vi "UHR-Fleezers Control (host) - 12.3.vi"() -> ()   [LabVIEW 2012] (continued)
                      n1986 = Square(x=w2941) -> (x^2=w2939:dbl)
                      n1987 = Square(x=w2940) -> (x^2=w2938:dbl)
                      n1988 = Add(x=w2939, y=w2938) -> (x+y=w2937:dbl)
                      n1989 = Square Root(x=w2937) -> (sqrt(x)=w2933:dbl)
                      n1990 = In Range and Coerce(upper limit="Limit Max (MHz)", x=w2933, lower limit="Limit Min (MHz)") -> (In Range?=w2926:bool)  [unwired: 1 out]
                      n1991 = Not(x="Limits Enable") -> (.not. x?=w2925:bool)
                      n1992 = Or(x=w2926, y=w2925) -> (x .or. y?=w2927:bool)
                      n1993 = case shown="True" w2927 {
                        tunnel: w2934 -> [_ w2967]
                        tunnel: w2933 -> [_ w2958]
                        tunnel: w2923 -> [_ w2965]
                        tunnel: w2932 -> [_ w2964]
                        tunnel: w2921 -> [_ w2963]
                        tunnel: w2931 -> [_ w2962]
                        tunnel: w2916 -> [_ w2960]
                        tunnel: w2915 -> [_ w2959]
                        frame False {
                        }
                        frame True {
                          n1994 = local read "BD 1 Frequency 3 (MHz)"() -> (w2966:dbl)
                          n1995 = local read "BD 2 Frequency 3 (MHz)"() -> (w2961:dbl)
                          n1996 = local write "Trap Delta (MHz)"(w2958) -> ()
                          n1997 = call "set RF board frequency - interlace.vi"("Board 2 Frequency Limits"=w2959, "Board 1 Frequency Limits"=w2960, "FPGA VI Reference In"=w2967, "Board 2 Frequency 3 (MHz)"=w2961, "Board 1 Frequency 3 (MHz)"=w2966, "Board 2 Frequency 2 (MHz)"=w2962, "Board 2 Frequency 1 (MHz)"=w2963, "Board 1 Frequency 2 (MHz)"=w2964, "Board 1 Frequency 1  (MHz)"=w2965) -> ()  [unwired: 1 in, 2 out]
                          n1998 = local write "BD 2 Frequency 1 (MHz)"(w2963) -> ()
                          n1999 = local write "BD 1 Frequency 1 (MHz)"(w2965) -> ()
                        }
                      }
                    }
                    frame True {
                    }
                  }
                }
                event Mouse Up {
                  n2000 = event-data() -> ("Button"=w2968:u16)  [unwired: 8 out]
                  n2001 = case shown="3" w2968 {
                    tunnel: [FALSE TRUE] -> w2969
                    frame 0, Default {
                    }
                    frame 3 {
                      n2002 = local read "Trap Delta (MHz)"() -> (w2971:dbl)
                      n2003 = property on="Initial delta (MHz)" class="DigNum (strict)"("Val(Sgnl)"=w2971) -> ()  [unwired: 2 in, 2 out]
                      n2004 = local write "Manipulating Trap"(FALSE ("Manipulating Trap")) -> ()
                    }
                  }
                }
              }
            }
          }
        }
      }
      event Mouse Move {
        n2005 = event-data() -> ()  [unwired: 6 out]
      }
    }
    n2006 = local read "Stop All"() -> (w2787:bool)
    n2007 = node-c288() -> ()  [unwired: 2 out]
  }
  n2008 = timed-loop "Main data acquisition loop (get data, process data for display, and save data to disk)" {
    tunnel: w7 -> [w3283]
    tunnel: w83 -> [w3282]
    tunnel: [w3312] -> w287
    tunnel: [w3307] -> w285
    timing: w195 -> [_]
    timing-out: [_] -> w194
    tunnel: w100 -> [w3136]
    stop <- "Stop All" stop-if-true
    w3053 = "Initialize"
    n2009 = node-c288() -> ()  [unwired: 2 out]
    n2010 = First Call?() -> (First Call?: T/F=w3088:bool)
    n2011 = Or(x="Reset", y=w3088) -> (x .or. y?=w3089:bool)
    n2012 = local read "Flushing P1"() -> (w3008:bool)
    n2013 = case "Reset data stream (manual reset or at begining of some rastering and imaging)" shown="True" w3089 {
      tunnel: w3283 -> [w4355 w4363]
      tunnel: w3282 -> [w4354 w4362]
      tunnel: [w4355 w4357] -> w3278
      tunnel: [w4354 w4356] -> w3277
      frame False {
      }
      frame True {
        w4360 = TRUE ("AI to FIFO")
        n2014 = local write "Overflow (data lost)"(FALSE ("Overflow (data lost)")) -> ()
        n2015 = call "reset FPGA DMA.vi"("error in"=w4362, "FPGA VI Reference In"=w4363) -> ("error out"=w4358:errorcluster, "FPGA VI Reference Out"=w4359:T19)
        n2016 = xnode "Read/Write Control"("FPGA VI Reference In"=w4359, "error in"=w4358, "AI to FIFO"=w4360, "APD to FIFO"=w4360) -> ("FPGA VI Reference Out"=w4357:T19, "error out"=w4356:errorcluster)
      }
    }
    n2017 = case shown="True" w3008 {
      frame False {
      }
      frame True {
        n2018 = local read "Flush rate (uL/m) P1"() -> (w3338:dbl)
        n2019 = local read "HP1 Flush Time (s)"() -> (w3347:dbl)
        n2020 = local read "DMA Update Period (s)"() -> (w3341:dbl)
        n2021 = Divide(x=w3338, y=60.0) -> (x/y=w3339:dbl)
        n2022 = Divide(x=w3347, y=w3341) -> (x/y=w3336:dbl)
        n2023 = feedback #1(0) -> (w3345:i32)
        n2024 = Increment(x=w3345) -> (x+1=w3335:i32)
        n2025 = Greater?(x=w3335, y=w3336) -> (0:w3344:bool)
        n2026 = Compound Arithmetic op=MULTIPLY(w3341, w3335, w3339) -> (→"P1 Flush Volume (uL)":dbl)
        n2027 = Divide(x=w3335, y=w3336) -> (x/y=→"P1 Flushing Bar":dbl)
        n2028 = case shown="True" w3344 {
          tunnel: w3335 -> [w3348 _]
          tunnel: [w3348 0] -> w3343
          frame False {
          }
          frame True {
            w3349 = FALSE ("Flushing P1")
            n2029 = local write "Inject Pump 1"(w3349) -> ()
            n2030 = local write "Flushing P1"(w3349) -> ()
            n2031 = property on="Clear Volume P1" class="Bool (strict)"("Val(Sgnl)"=TRUE ("Value (Signaling)")) -> ()  [unwired: 2 in, 2 out]
          }
        }
        n2032 = feedback-in #1(w3343) -> ()
      }
    }
    n2033 = Or(x="Start AOD Scan", y="Trap Raster Scan") -> (x .or. y?=w3234:bool)
    n2034 = case "Start AOM raster scan" shown="True" w3234 {
      tunnel: w3278 -> [w4205 w4215]
      tunnel: w3277 -> [w4204 w4214]
      tunnel: [w4205 w4208] -> w3276
      tunnel: [w4204 w4207] -> w3275
      frame False {
      }
      frame True {
        n2035 = case shown="True" "Restart DMA? (AOD)" {
          tunnel: [w4253 w4255] -> w4209
          tunnel: [w4252 w4254] -> w4210
          tunnel: w4215 -> [w4253 w4257]
          tunnel: w4214 -> [w4252 w4256]
          frame False {
          }
          frame True {
            n2036 = local write "Overflow (data lost)"(FALSE ("Overflow (data lost)")) -> ()
            n2037 = call "reset FPGA DMA.vi"("error in"=w4256, "FPGA VI Reference In"=w4257) -> ("error out"=w4254:errorcluster, "FPGA VI Reference Out"=w4255:T19)
          }
        }
        n2038 = local write "Trap Raster Scan"(FALSE ("Trap Raster Scan")) -> ()
        n2039 = case shown="True" "Move MCL Also?" {
          tunnel: w4210 -> [w4218 w4247]
          tunnel: w4209 -> [w4219 w4248]
          tunnel: [w4217 w4251] -> w4208
          tunnel: [w4216 w4250] -> w4207
          frame False {
            w4220 = TRUE ("AI to FIFO")
            n2040 = xnode "Read/Write Control"("FPGA VI Reference In"=w4219, "error in"=w4218, "AI to FIFO"=w4220, "APD to FIFO"=w4220, "Start scan"=w4220) -> ("FPGA VI Reference Out"=w4217:T19, "error out"=w4216:errorcluster)
          }
          frame True {
            w4244 = FALSE ("1D or 2D Scan?")
            w4249 = TRUE ("AI to FIFO")
            # "Count for MCL loop"
            # "N total cycles"
            # "N steps"
            # "V_int"
            n2041 = local read "Scan Range (nm)"() -> (w4226:dbl)
            n2042 = local read "Number of F/B Scans (AOD)"() -> (w4243:u16)
            n2043 = Sign(1:w4226) -> (0:w4225:dbl)
            n2044 = Compound Arithmetic op=MULTIPLY(w4226, "MCL Step Position Ratio", "MCL/AOM Scale Tweak") -> (w4230:dbl)
            n2045 = Negate(x=w4225) -> (-x=w4222:dbl)
            n2046 = Multiply(x=w4222, y="MCL Step Increment (V_int)") -> (x*y=w4224:dbl)
            n2047 = Divide(x=w4230, y="MCL X Cal (nm/V)") -> (x/y=w4236:dbl)
            n2048 = Multiply(x=32767.0 ("y"), y=w4236) -> (x*y=w4242:dbl)
            n2049 = local read "Total Counts (ticks)"() -> (w4227:u16)
            n2050 = local read "Cycles/step (AOD)"() -> (w4238:u64)
            n2051 = local read "Scan steps (AOD)"() -> (w4239:u64)
            n2052 = Divide(x=w4242, y=10.0) -> (x/y=w4235:dbl)
            n2053 = Divide(x=w4235, y="MCL Step Increment (V_int)") -> (x/y=w4233:dbl)
            n2054 = Absolute Value(x=w4233) -> (abs(x)=w4221:dbl)
            n2055 = Compound Arithmetic op=MULTIPLY(w4239, w4238, w4227) -> (w4234:u64)
            n2056 = local write "wait to reset values"(w4249) -> ()
            n2057 = local write "MCL Scanning"(w4249) -> ()
            n2058 = Divide(x=w4234, y=w4221) -> (x/y=w4231:dbl)
            "MCL Count" <- w4231
            n2059 = xnode "Read/Write Control"("FPGA VI Reference In"=w4248, "error in"=w4247, "Scan steps (MCL)"=w4221, "Number of scans (MCL)"=w4243, "Cycles per step (MCL)"=u64 1, "Scan freq.  increment (MCL)"=w4224, "1D or 2D Scan?"=w4244, "MCL Scan Axis"=w4244, "Cont. Scan (MCL)"=w4244, "MCL count"=w4231) -> ("FPGA VI Reference Out"=w4246:T19, "error out"=w4245:errorcluster)
            n2060 = xnode "Read/Write Control"("FPGA VI Reference In"=w4246, "error in"=w4245, "AI to FIFO"=w4249, "APD to FIFO"=w4249, "Start scan"=w4249, "Start scan (MCL)"=w4249) -> ("FPGA VI Reference Out"=w4251:T19, "error out"=w4250:errorcluster)
          }
        }
        "Raster Scanning..." <- TRUE ("Scanning...")
      }
    }
    n2061 = local read "Flushing P3"() -> (w3009:bool)
    n2062 = case "Keep track of when Harvard Pump 3 is done flushing" shown="True" w3009 {
      frame False {
      }
      frame True {
        n2063 = local read "Flush rate (uL/m) P3"() -> (w3355:dbl)
        n2064 = local read "DMA Update Period (s)"() -> (w3357:dbl)
        n2065 = local read "HP3 Flush Time (s)"() -> (w3364:dbl)
        n2066 = Divide(x=w3355, y=60.0) -> (x/y=w3353:dbl)
        n2067 = feedback #2(0) -> (w3362:i32)
        n2068 = Increment(x=w3362) -> (x+1=w3356:i32)
        n2069 = Divide(x=w3364, y=w3357) -> (x/y=w3358:dbl)
        n2070 = Greater?(x=w3356, y=w3358) -> (0:w3361:bool)
        n2071 = Compound Arithmetic op=MULTIPLY(w3357, w3356, w3353) -> (→"P3 Flush Volume (uL)":dbl)
        n2072 = case shown="True" w3361 {
          tunnel: w3356 -> [w3365 _]
          tunnel: [w3365 0] -> w3360
          frame False {
          }
          frame True {
            w3366 = FALSE ("Flushing P3")
            n2073 = local write "Inject Pump 3"(w3366) -> ()
            n2074 = local write "Flushing P3"(w3366) -> ()
            n2075 = property on="Clear Volume P3" class="Bool (strict)"("Val(Sgnl)"=TRUE ("Value (Signaling)")) -> ()  [unwired: 2 in, 2 out]
          }
        }
        n2076 = feedback-in #2(w3360) -> ()
        n2077 = Divide(x=w3356, y=w3358) -> (x/y=→"P3 Flushing Bar":dbl)
      }
    }
    n2078 = And(x="Save scans", y=w3234) -> (x .and. y?=w3274:bool)
    n2079 = Compound Arithmetic op=OR("Start MCL Scan", "Confocal Image", "Confocal Linescan") -> (w3232:bool)
    n2080 = And(x="Save Data (MCL)", y=w3232) -> (x .and. y?=w3273:bool)
    n2081 = case "Start MCL raster scan" shown="True" w3232 {
      tunnel: w3276 -> [w3817 w3833]
      tunnel: w3275 -> [w3816 w3832]
      tunnel: [w3817 w3828] -> w3135
      tunnel: [w3816 w3827] -> w3134
      tunnel: [FALSE w3826] -> w3259
      tunnel: "Start MCL Scan" -> [_ w3821]
      tunnel: "Confocal Image" -> [_ w3820]
      tunnel: "Confocal Linescan" -> [_ _]
      frame False {
      }
      frame True {
        w3826 = TRUE
        n2082 = case shown="True" "Restart DMA? (MCL)" {
          tunnel: [w3878 w3880] -> w3831
          tunnel: [w3877 w3879] -> w3830
          tunnel: w3833 -> [w3878 w3883]
          tunnel: w3832 -> [w3877 w3882]
          frame False {
          }
          frame True {
            n2083 = call "reset FPGA DMA.vi"("error in"=w3882, "FPGA VI Reference In"=w3883) -> ("error out"=w3879:errorcluster, "FPGA VI Reference Out"=w3880:T19)
            n2084 = local write "Overflow (data lost)"(FALSE ("Overflow (data lost)")) -> ()
          }
        }
        n2085 = case shown="False" w3821 {
          selector: w3821 -> [_ w3837]
          tunnel: w3820 -> [w3836 _]
          tunnel: [w3836 w3837] -> w3819
          frame False {
            n2086 = property on="2D or 1D Scan" class="Bool (strict)"("Val(Sgnl)"=w3836) -> ()  [unwired: 2 in, 2 out]
            n2087 = property on="Confocal Image" class="Bool (strict)"("Value"=FALSE ("Start Confocal Map")) -> ()  [unwired: 2 in, 2 out]
          }
          frame True {
          }
        }
        n2088 = local write "MCL Scanning"(w3826) -> ()
        n2089 = local read "AO1"() -> (w3823:dbl)
        n2090 = local read "AO2"() -> (w3822:dbl)
        n2091 = case shown="True" "Center Scan" {
          tunnel: w3831 -> [w3844 w3876]
          tunnel: w3830 -> [w3843 w3875]
          tunnel: [w3842 w3874] -> w3828
          tunnel: [w3841 w3873] -> w3827
          tunnel: [w3839 w3860] -> w3825
          tunnel: [w3838 w3859] -> w3824
          tunnel: w3823 -> [w3839 w3865]
          tunnel: w3822 -> [w3838 w3868]
          tunnel: w3819 -> [_ _]
          frame False {
            w3840 = TRUE ("AI to FIFO")
            n2092 = xnode "Read/Write Control"("FPGA VI Reference In"=w3844, "error in"=w3843, "AI to FIFO"=w3840, "APD to FIFO"=w3840, "Start scan (MCL)"=w3840) -> ("FPGA VI Reference Out"=w3842:T19, "error out"=w3841:errorcluster)
          }
          frame True {
            w3872 = TRUE ("AI to FIFO")
            n2093 = local read "Scan steps (MCL)"() -> (w3851:u64)
            n2094 = local read "Scan lines (y)"() -> (w3847:u64)
            n2095 = local read "Fast Scan Dir"() -> (w3858:bool)
            n2096 = local read "Actual MCL Inc (V)"() -> (w3848:dbl)
            n2097 = Decrement(x=w3847) -> (x-1=w3846:u64)
            n2098 = Decrement(x=w3851) -> (x-1=w3850:u64)
            n2099 = Multiply(x=w3848, y=w3846) -> (x*y=w3845:dbl)
            n2100 = Divide(x=w3845, y=2.0) -> (x/y=w3855:dbl)
            n2101 = Multiply(x=w3848, y=w3850) -> (x*y=w3849:dbl)
            n2102 = Divide(x=w3849, y=2.0) -> (x/y=w3854:dbl)
            n2103 = Select(t=w3854, s=w3858, f=w3855) -> (s? t:f=w3853:dbl)
            n2104 = Select(t=w3855, s=w3858, f=w3854) -> (s? t:f=w3857:dbl)
            n2105 = Subtract(x=w3865, y=w3857) -> (x-y=w3856:dbl)
            n2106 = Subtract(x=w3868, y=w3853) -> (x-y=w3852:dbl)
            n2107 = local read "2D or 1D Scan"() -> (w3870:bool)
            n2108 = Not(x=w3858) -> (.not. x?=w3864:bool)
            n2109 = Not(x=w3870) -> (.not. x?=w3866:bool)
            n2110 = And(x=w3858, y=w3866) -> (x .and. y?=w3867:bool)
            n2111 = And(x=w3866, y=w3864) -> (x .and. y?=w3869:bool)
            n2112 = Select(t=w3868, s=w3869, f=w3852) -> (s? t:f=w3859:dbl)
            n2113 = Select(t=w3865, s=w3867, f=w3856) -> (s? t:f=w3860:dbl)
            n2114 = call "Volt to I16.vi"("Voltage In"=w3860) -> ("I16 Voltage Out"=w3863:i16)
            n2115 = call "Volt to I16.vi"("Voltage In"=w3859) -> ("I16 Voltage Out"=w3862:i16)
            n2116 = xnode "Read/Write Control"("FPGA VI Reference In"=w3876, "error in"=w3875, "AI to FIFO"=w3872, "APD to FIFO"=w3872, "Start scan (MCL)"=w3872, "AO1"=w3863, "AO2"=w3862) -> ("FPGA VI Reference Out"=w3874:T19, "error out"=w3873:errorcluster)
          }
        }
        "Initial Y" <- w3825
        "Initial X" <- w3824
        n2117 = local write "Tab Control 6"(T3."Imaging" ("Tab Control 6")) -> ()
        "wait to reset values" <- w3826
      }
    }
    n2118 = local read "APD Elements/DMA read"() -> (w2974:u32)
    n2119 = local read "Trap AI Elements/DMA read"() -> (w3197:u32)
    n2120 = xnode "Get APD Data"("FPGA VI Reference In"=w3135, "error in"=w3134, "Number of Elements"=w2974, "Timeout (ms)"=-1) -> ("Data"=w3166:u32[], "Elements Remaining"=→"APD FIFO Elements Remaining":u32)  [unwired: 2 out]
    n2121 = local read "Trap Pos Elements/DMA read"() -> (w3131:u32)
    n2122 = xnode "Invoke Method"("FPGA VI Reference In"=w3135, "error in"=w3134, "Number of Elements"=w3131, "Timeout (ms)"=-1) -> ("Data"=w3095:u16[], "Elements Remaining"=→"Trap Pos FIFO El Remaining":u32)  [unwired: 2 out]
    n2123 = xnode "Get Trap Data"("FPGA VI Reference In"=w3135, "error in"=w3134, "Number of Elements"=w3197, "Timeout (ms)"=-1 ("Timeout")) -> ("FPGA VI Reference Out"=w3030:T19, "error out"=w3029:errorcluster, "Data"=w3096:i16[], "Elements Remaining"=w3320:u32)
    "FIFO El. Rem." <- w3320
    n2124 = local read "DMA Update Period (s)"() -> (w3198:dbl)
    n2125 = local read "Trap AI FIFO Depth"() -> (w3322:u32)
    n2126 = local read "Number of APDs"() -> (w2998:u8)
    n2127 = Decimate 1D Array(w3095) -> (w3092:u16[], w3094:u16[], w3093:u16[])
    n2128 = feedback #3(0.0) -> (w3124:dbl)
    n2129 = Add(x=w3198, y=w3124) -> (x+y=w3296:dbl)
    n2130 = feedback-in #3(w3296) -> ()
    n2131 = To Time Stamp(1:w3124) -> (0:w3123:timestamp)
    n2132 = Subtract(x=w3322, y=w3197) -> (x-y=w3321:u32)
    n2133 = To Unsigned Long Integer(number=w3092) -> (unsigned 32bit integer=w3091:u32[])
    n2134 = Join Numbers(hi=w3094, lo=w3093) -> ((hi.lo)=w3090:u32[])
    n2135 = Divide(x=w3320, y=w3321) -> (x/y=w3319:dbl)
    "Buffer Status" <- w3319
    n2136 = case "Deinterlace APD signals" shown="2" w2998 {
      tunnel: [w3328 w3334] -> w2981
      tunnel: w3166 -> [w3329 w3333]
      tunnel: [w3327 w3332] -> w2980
      tunnel: [w3326 w3330] -> w2979
      frame 3, Default {
        n2137 = Decimate 1D Array "APD signals"(w3329) -> (w3328:u32[], w3327:u32[], w3326:u32[])
      }
      frame 2 {
        n2138 = Decimate 1D Array "APD signals"(w3333) -> (w3334:u32[], w3332:u32[])
        n2139 = Multiply(x=w3332, y=u32 0) -> (x*y=w3330:u32[])
      }
    }
    n2140 = Join Numbers(hi=w3091, lo=w3090) -> ((hi.lo)=w3084:u64[])
    n2141 = call "IR AOM word to freq - vec.vi"("Frequency Word In (double vec)"=w3084) -> ("Frequency Out"=w3130:dbl[])
    n2142 = Equal?(x=w3319, y=1.0) -> (x = y?=w3317:bool)
    n2143 = case "Alert buffer overflow" shown="True" w3317 {
      frame False {
      }
      frame True {
        n2144 = call <vilib>:"Beep.vi"() -> ()  [unwired: 3 in, 9 out]
        "Overflow (data lost)" <- TRUE ("Overflow (data lost)")
      }
    }
    n2145 = Decimate 1D Array(w3130) -> (w3129:dbl[], w3128:dbl[])
    n2146 = Build Array(w3129, w3128) -> (w3127:dbl[][])
    n2147 = Build Array(w2981, w2980, w2979) -> (w3256:u32[][])
    n2148 = Bundle(w2981, w2980, w2979) -> (w2977:cluster{u32[], u32[], u32[]})  [unwired: 1 in]
    n2149 = local read "APD Integration Time (s)"() -> (w2991:dbl)
    n2150 = To Double Precision Float(number=w3256) -> (double precision float=w3257:dbl[][])
    n2151 = feedback #4 "APD3"(w2979) -> (w2997:u32[])
    n2152 = feedback #5 "APD2"(w2980) -> (w3153:u32[])
    n2153 = feedback #6 "APD1"(w2981) -> (w3255:u32[])
    n2154 = Build Array (concatenate)(w3153, w2980) -> (w3152:u32[])
    n2155 = Build Array (concatenate)(w2997, w2979) -> (w2996:u32[])
    n2156 = Build Array (concatenate)(w3255, w2981) -> (w3252:u32[])
    n2157 = Array Size(array=w3252) -> (size(s)=w3249:i32)
    n2158 = Array Size(array=w2981) -> (size(s)=w3251:i32)
    n2159 = Multiply(x=w3251, y="APD Ave N") -> (x*y=w3250:dbl)
    n2160 = Greater?(x=w3249, y=w3250) -> (0:w3253:bool)
    n2161 = Bundle("APD 1", "APD 2", "APD 3") -> (w3289:cluster{string, string, string})  [unwired: 1 out]
    n2162 = local read "Trap Sets"() -> (w3196:u32)
    n2163 = case shown="True" w3253 {
      tunnel: w3252 -> [w3632 w3641]
      tunnel: [w3632 w3639] -> w3203
      tunnel: w3250 -> [_ w3634]
      tunnel: w3249 -> [_ w3640]
      tunnel: w3152 -> [w3631 w3638]
      tunnel: [w3631 w3637] -> w3150
      tunnel: w2996 -> [w3630 w3636]
      tunnel: [w3630 w3633] -> w2992
      frame False {
      }
      frame True {
        n2164 = Subtract(x=w3640, y=w3634) -> (x-y=w3635:dbl)
        n2165 = Array Subset "APD3"(array=w3636, index=w3635, length=w3634) -> (w3633:u32[])
        n2166 = Array Subset "APD2"(array=w3638, index=w3635, length=w3634) -> (w3637:u32[])
        n2167 = Array Subset "APD1"(array=w3641, index=w3635, length=w3634) -> (w3639:u32[])
      }
    }
    n2168 = feedback-in #4(w2992) -> ()
    n2169 = feedback-in #5(w3150) -> ()
    n2170 = feedback-in #6(w3203) -> ()
    n2171 = Cluster To Array(cluster=w3289) -> (array=w3286:string[])
    n2172 = for "APD" {
      tunnel: w3257 -> [w3888] mode=indexing
      tunnel: w2991 -> [w3895]
      tunnel: [w3891] -> w3154 mode=indexing
      tunnel: "APD Disp. Scale" -> [w3892]
      tunnel: w3286 -> [w3890] mode=indexing
      tunnel: "APD Disp. Downsample" -> [w3886]
      tunnel: [w3889] -> w3285
      workers-P: _ -> [_]
      tunnel: w3123 -> [w3885]
      n2173 = call "integrate 1D array interval - double.vi"("Ave N"=w3886, "Array In"=w3888) -> ("Array Out"=w3887:dbl[])  [unwired: 1 out]
      n2174 = Multiply(x=w3895, y=w3886) -> (x*y=w3889:dbl)
      n2175 = Divide(x=w3887, y=w3892) -> (x/y=w3893:dbl[])
      n2176 = Bundle By Name("t0"=w3885, "Y"=w3893, "dt"=w3889) -> (w3894:waveform(dbl))  [unwired: 1 out]
      n2177 = Set Waveform Attribute(5:w3890, 6:"NI_ChannelName" ("name"), 7:w3894) -> (3:w3891:waveform(dbl))  [unwired: 1 in, 2 out]
    }
    "APD Display Period (s)" <- w3285
    n2178 = Reciprocal(x=w3285) -> (1/x=→"APD Display Freq. (Hz)":dbl)
    n2179 = case "Deinterlace trap data, average down PSD" shown="2" w3196 {
      tunnel: w3096 -> [w3913 w3978]
      tunnel: [w3910 w3975] -> w3189
      tunnel: [w3913 w3977] -> w3087
      tunnel: "Detector Type" -> [w3912 w3973]
      tunnel: [w3911 w3976] -> w3188
      tunnel: [w3909 w3974] -> w3294
      frame 1, Default {
        n2180 = Divide(x=w3913, y=3276.7) -> (x/y=w3914:dbl[])
        n2181 = Decimate 1D Array(w3914) -> (w3923:dbl[], w3922:dbl[], w3921:dbl[], w3920:dbl[], w3919:dbl[], w3918:dbl[], w3917:dbl[], w3916:dbl[])
        n2182 = case shown="\"IR-QPD + PSD + FB-QPD position\"" w3912 {
          tunnel: w3923 -> [w3947 w3972]
          tunnel: w3922 -> [w3946 w3971]
          tunnel: w3921 -> [w3931 w3949]
          tunnel: w3920 -> [w3932 w3959]
          tunnel: w3919 -> [w3945 w3970]
          tunnel: w3918 -> [w3944 w3969]
          tunnel: w3917 -> [w3928 w3950]
          tunnel: w3916 -> [w3927 w3948]
          tunnel: [w3926 w3956] -> w3911
          tunnel: [w3925 w3955] -> w3910
          tunnel: [w3924 w3954] -> w3909
          frame "IR-QPD + PSD + FB-QPD", Default {
            w3924 = 0  # Channel pattern
            n2183 = Divide(x=w3947, y=w3932) -> (x/y=w3934:dbl[])
            n2184 = Divide(x=w3946, y=w3932) -> (x/y=w3933:dbl[])
            n2185 = Divide(x=w3945, y=w3928) -> (x/y=w3930:dbl[])
            n2186 = Divide(x=w3944, y=w3927) -> (x/y=w3929:dbl[])
            n2187 = Build Array(w3934, w3933, w3932, w3931, w3930, w3929, w3928, w3927) -> (w3925:dbl[][])
            n2188 = Bundle("T1 Y", "T1 X", "T1 Sum", "FB Sum", "PSD Y", "PSD X", "PSD Y Sum", "PSD X Sum") -> (w3943:T38)  [unwired: 1 out]
            n2189 = Cluster To Array(cluster=w3943) -> (array=w3926:string[])
          }
          frame "IR-QPD + PSD + FB-QPD position" {
            w3954 = 3  # Channel pattern
            n2190 = Negate(x=w3950) -> (-x=w3951:dbl[])
            n2191 = Divide(x=w3972, y=w3959) -> (x/y=w3961:dbl[])
            n2192 = Divide(x=w3971, y=w3959) -> (x/y=w3960:dbl[])
            n2193 = Divide(x=w3970, y=w3950) -> (x/y=w3958:dbl[])
            n2194 = Divide(x=w3969, y=w3951) -> (x/y=w3957:dbl[])
            n2195 = Build Array(w3961, w3960, w3959, w3948, w3949, w3958, w3957, w3950) -> (w3955:dbl[][])
            n2196 = Bundle("T1 Y", "T1 X", "T1 Sum", "FB X", "FB Sum", "PSD Y", "PSD X", "PSD Y Sum") -> (w3968:T38)  [unwired: 1 out]
            n2197 = Cluster To Array(cluster=w3968) -> (array=w3956:string[])
          }
        }
      }
      frame 2 {
        n2198 = case shown="\"IR-QPD + PSD + FB-QPD X position\"" w3973 {
          tunnel: w3978 -> [w4040 w4112 w4183]
          tunnel: [w3979 w4103 w4114] -> w3977
          tunnel: [w4006 w4094 w4161] -> w3976
          tunnel: [w4005 w4057 w4128] -> w3975
          tunnel: [w3999 w4092 w4159] -> w3974
          frame "IR-QPD + PSD + FB-QPD", Default {
            w3999 = 1  # Channel pattern
            # "time average x2 the 4th signal and the 4 psd signals (detection laser)"
            # "deinterlace 3 signals from qpd"
            n2199 = Decimate 1D Array(w4040) -> (w4039:i16[], w4038:i16[], w4004:i16[], w4037:i16[], w4027:i16[], w4025:i16[], w4024:i16[], w4022:i16[])
            n2200 = Decimate 1D Array(w4004) -> (w4003:i16[], w4002:i16[])
            n2201 = Decimate 1D Array(w4039) -> (w4036:i16[], w4008:i16[])
            n2202 = Decimate 1D Array(w4038) -> (w4035:i16[], w4033:i16[])
            n2203 = Decimate 1D Array(w4037) -> (w4034:i16[], w4032:i16[])
            n2204 = call "downsample 1D array - double.vi"("Ave N"=2.0, "Array In"=w4027) -> ("Array Out"=w4026:dbl[])  [unwired: 1 out]
            n2205 = call "downsample 1D array - double.vi"("Ave N"=2.0, "Array In"=w4025) -> ("Array Out"=w4007:dbl[])  [unwired: 1 out]
            n2206 = call "downsample 1D array - double.vi"("Ave N"=2.0, "Array In"=w4024) -> ("Array Out"=w4023:dbl[])  [unwired: 1 out]
            n2207 = call "downsample 1D array - double.vi"("Ave N"=2.0, "Array In"=w4022) -> ("Array Out"=w4021:dbl[])  [unwired: 1 out]
            n2208 = Interleave 1D Arrays(w4036, w4035, w4034, w4008, w4033, w4032, w4003, w4002, w4026, w4007, w4023, w4021) -> (w4020:dbl[])
            n2209 = Divide(x=w4020, y=3276.7) -> (x/y=w4019:dbl[])
            n2210 = Decimate 1D Array(w4019) -> (w4018:dbl[], w4017:dbl[], w4016:dbl[], w4015:dbl[], w4014:dbl[], w4013:dbl[], w4001:dbl[], w4000:dbl[], w4012:dbl[], w4011:dbl[], w4010:dbl[], w4009:dbl[])
            n2211 = Divide(x=w4018, y=w4016) -> (x/y=w3986:dbl[])
            n2212 = Divide(x=w4017, y=w4016) -> (x/y=w3985:dbl[])
            n2213 = Divide(x=w4015, y=w4013) -> (x/y=w3984:dbl[])
            n2214 = Divide(x=w4014, y=w4013) -> (x/y=w3983:dbl[])
            n2215 = Divide(x=w4012, y=w4010) -> (x/y=w3982:dbl[])
            n2216 = Divide(x=w4011, y=w4009) -> (x/y=w3981:dbl[])
            n2217 = Build Array(w3986, w3985, w4016, w3984, w3983, w4013, w4001, w4000, w3982, w3981, w4010, w4009) -> (w4005:dbl[][])
            n2218 = Bundle("T1 Y", "T1 X", "T1 Sum", "T2 Y", "T2 X", "T2 Sum", "T1 FB Sum", "T2 FB Sum", "PSD Y", "PSD X", "PSD Y Sum", "PSD X Sum") -> (w3987:T39)  [unwired: 1 out]
            n2219 = To Word Integer(number=w4020) -> (16bit integer=w3979:i16[])
            n2220 = Cluster To Array(cluster=w3987) -> (array=w4006:string[])
          }
          frame "IR-QPD + PSD + FB-QPD X position" {
            w4092 = 2  # Channel pattern
            # "time average x2 the 3 psd signals (detection laser)"
            # "deinterlace 3 signals from qpds"
            n2221 = Decimate 1D Array(w4112) -> (w4111:i16[], w4110:i16[], w4093:i16[], w4109:i16[], w4055:i16[], w4052:i16[], w4049:i16[], w4080:i16[])
            n2222 = Select(t=i16 -1, s="Flip X Sign", f=i16 1) -> (s? t:f=w4045:i16)
            n2223 = Multiply(x=w4110, y=w4045) -> (x*y=w4046:i16[])
            n2224 = Decimate 1D Array(w4093) -> (w4078:i16[], w4076:i16[])
            n2225 = Decimate 1D Array(w4111) -> (w4108:i16[], w4095:i16[])
            n2226 = Decimate 1D Array(w4046) -> (w4107:i16[], w4105:i16[])
            n2227 = Decimate 1D Array(w4109) -> (w4106:i16[], w4104:i16[])
            n2228 = Decimate 1D Array(w4080) -> (w4079:i16[], w4077:i16[])
            n2229 = call "downsample 1D array - I16.vi"("Ave N"=2.0, "Array In"=w4055) -> ("Array Out"=w4053:i16[])  [unwired: 1 in]
            n2230 = call "downsample 1D array - I16.vi"("Ave N"=2.0, "Array In"=w4049) -> ("Array Out"=w4047:i16[])  [unwired: 1 in]
            n2231 = call "downsample 1D array - I16.vi"("Ave N"=2.0, "Array In"=w4052) -> ("Array Out"=w4050:i16[])  [unwired: 1 in]
            n2232 = Interleave 1D Arrays(w4108, w4107, w4106, w4095, w4105, w4104, w4079, w4078, w4077, w4076, w4053, w4050, w4047) -> (w4103:i16[])
            n2233 = Divide(x=w4103, y=3276.7) -> (x/y=w4102:dbl[])
            n2234 = Decimate 1D Array(w4102) -> (w4101:dbl[], w4100:dbl[], w4099:dbl[], w4098:dbl[], w4097:dbl[], w4096:dbl[], w4068:dbl[], w4066:dbl[], w4065:dbl[], w4063:dbl[], w4062:dbl[], w4061:dbl[], w4058:dbl[])
            n2235 = Negate(x=w4058) -> (-x=w4056:dbl[])
            n2236 = Divide(x=w4062, y=w4058) -> (x/y=w4060:dbl[])
            n2237 = Divide(x=w4061, y=w4056) -> (x/y=w4059:dbl[])
            n2238 = Divide(x=w4101, y=w4099) -> (x/y=w4084:dbl[])
            n2239 = Divide(x=w4100, y=w4099) -> (x/y=w4083:dbl[])
            n2240 = Divide(x=w4098, y=w4096) -> (x/y=w4082:dbl[])
            n2241 = Divide(x=w4097, y=w4096) -> (x/y=w4081:dbl[])
            n2242 = Divide(x=w4068, y=w4066) -> (x/y=w4067:dbl[])
            n2243 = Divide(x=w4065, y=w4063) -> (x/y=w4064:dbl[])
            n2244 = Build Array(w4084, w4083, w4099, w4082, w4081, w4096, w4067, w4066, w4064, w4063, w4060, w4059, w4058) -> (w4057:dbl[][])
            n2245 = Bundle("T1 Y", "T1 X", "T1 Sum", "T2 Y", "T2 X", "T2 Sum", "T1 FB X", "T1 FB Sum", "T2 FB X", "T2 FB Sum", "PSD Y", "PSD X", "PSD Y Sum") -> (w4085:T40)  [unwired: 1 out]
            n2246 = Cluster To Array(cluster=w4085) -> (array=w4094:string[])
          }
          frame "IR-QPD + PSD + FB-QPD XY positions" {
            w4159 = 4  # Channel pattern
            # "time average x2 the 3 psd signals (detection laser)"
            # "deinterlace 3 signals from qpds"
            n2247 = Decimate 1D Array(w4183) -> (w4182:i16[], w4181:i16[], w4160:i16[], w4180:i16[], w4126:i16[], w4172:i16[], w4171:i16[], w4148:i16[])
            n2248 = Decimate 1D Array "Feedback Sum"(w4160) -> (w4144:i16[], w4142:i16[])
            n2249 = Decimate 1D Array "QPD Y"(w4182) -> (w4179:i16[], w4162:i16[])
            n2250 = Decimate 1D Array "QPD X"(w4181) -> (w4178:i16[], w4176:i16[])
            n2251 = Decimate 1D Array "Feedback Y"(w4126) -> (w4125:i16[], w4124:i16[])
            n2252 = Decimate 1D Array "QPD Sum"(w4180) -> (w4177:i16[], w4175:i16[])
            n2253 = Decimate 1D Array "Feedback X"(w4148) -> (w4145:i16[], w4143:i16[])
            n2254 = call "downsample 1D array - double.vi"("Ave N"=2.0, "Array In"=w4172) -> ("Array Out"=w4147:dbl[])  [unwired: 1 out]
            n2255 = call "downsample 1D array - double.vi"("Ave N"=2.0, "Array In"=w4171) -> ("Array Out"=w4146:dbl[])  [unwired: 1 out]
            n2256 = Interleave 1D Arrays(w4179, w4178, w4177, w4162, w4176, w4175, w4125, w4145, w4144, w4124, w4143, w4142, w4147, w4146) -> (w4170:dbl[])
            n2257 = Divide(x=w4170, y=3276.7) -> (x/y=w4169:dbl[])
            n2258 = Decimate 1D Array(w4169) -> (w4168:dbl[], w4167:dbl[], w4166:dbl[], w4165:dbl[], w4164:dbl[], w4163:dbl[], w4121:dbl[], w4135:dbl[], w4119:dbl[], w4120:dbl[], w4133:dbl[], w4117:dbl[], w4131:dbl[], w4129:dbl[])
            n2259 = Negate(x=w4129) -> (-x=w4127:dbl[])
            n2260 = Divide(x=w4131, y=w4127) -> (x/y=w4130:dbl[])
            n2261 = Divide(x=w4120, y=w4117) -> (x/y=w4116:dbl[])
            n2262 = Divide(x=w4121, y=w4119) -> (x/y=w4118:dbl[])
            n2263 = Divide(x=w4168, y=w4166) -> (x/y=w4152:dbl[])
            n2264 = Divide(x=w4167, y=w4166) -> (x/y=w4151:dbl[])
            n2265 = Divide(x=w4165, y=w4163) -> (x/y=w4150:dbl[])
            n2266 = Divide(x=w4164, y=w4163) -> (x/y=w4149:dbl[])
            n2267 = Divide(x=w4135, y=w4119) -> (x/y=w4134:dbl[])
            n2268 = Divide(x=w4133, y=w4117) -> (x/y=w4132:dbl[])
            n2269 = Build Array(w4152, w4151, w4166, w4150, w4149, w4163, w4118, w4134, w4119, w4116, w4132, w4117, w4130, w4129) -> (w4128:dbl[][])
            n2270 = Bundle("T1 Y", "T1 X", "T1 Sum", "T2 Y", "T2 X", "T2 Sum", "T1 FB Y", "T1 FB X", "T1 FB Sum", "T2 FB Y", "T2 FB X", "T2 FB Sum", "PSD X", "PSD Y Sum") -> (w4115:T41)  [unwired: 1 out]
            n2271 = To Word Integer(number=w4170) -> (16bit integer=w4114:i16[])
            n2272 = Cluster To Array(cluster=w4115) -> (array=w4161:string[])
          }
        }
      }
    }
    "AI labels" <- w3188
    n2273 = local read "APD Integration Time (s)"() -> (w3161:dbl)
    n2274 = Array Size(array=w3203) -> (size(s)=w3248:i32)
    n2275 = call <vilib>:"Std Deviation and Variance.vi"("X"=w3150) -> ("standard deviation"=w3149:dbl)  [unwired: 1 in, 2 out]
    n2276 = Add Array Elements(numeric array=w3150) -> (sum=w3151:u32)
    n2277 = Add Array Elements(numeric array=w3203) -> (sum=w3258:u32)
    n2278 = call <vilib>:"Std Deviation and Variance.vi"("X"=w3203) -> ("standard deviation"=w3202:dbl)  [unwired: 1 in, 2 out]
    n2279 = Divide(x=w3149, y=w2991) -> (x/y=w3146:dbl)
    "Rate sigma (Hz) 2" <- w3146
    n2280 = Multiply(x=w2991, y=w3248) -> (x*y=w2993:dbl)
    "Int. Time (s)" <- w2993
    n2281 = Divide(x=w3151, y=w2993) -> (x/y=w3147:dbl)
    "APD 2 Rate (Hz)" <- w3147
    n2282 = Multiply(x="APD Disp. Scale", y=w3154) -> (x*y=w3163:waveform(dbl)[])
    n2283 = Divide(x=w3258, y=w2993) -> (x/y=w3200:dbl)
    "APD 1 Rate (Hz)" <- w3200
    n2284 = Divide(x=w3202, y=w2991) -> (x/y=w3201:dbl)
    "Rate sigma (Hz)" <- w3201
    n2285 = Divide(x=w3146, y=w3147) -> (x/y=→"Sigma/Mean 2":dbl)
    n2286 = Multiply(x="APD Disp. Downsample", y=w3161) -> (x*y=w3159:dbl)
    n2287 = Divide(x=w3201, y=w3200) -> (x/y=→"Sigma/Mean":dbl)
    n2288 = Divide(x=w3163, y=w3159) -> (x/y=w2983:waveform(dbl)[])
    n2289 = Index Array(array=w2983, index=0) -> (element=w3143:waveform(dbl))
    n2290 = Index Array(array=w2983, index=1) -> (element=w3141:waveform(dbl))
    n2291 = Index Array(array=w2983, index=2) -> (element=w2985:waveform(dbl))
    n2292 = Subtract(x=w3143, y="APD 1 Offset") -> (x-y=w3139:waveform(dbl))
    n2293 = Subtract(x=w3141, y="APD 2 Offset") -> (x-y=w3138:waveform(dbl))
    n2294 = Subtract(x=w2985, y="APD 3 Offset") -> (x-y=w2982:waveform(dbl))
    n2295 = Add Array Elements(numeric array=w2992) -> (sum=w2995:u32)
    n2296 = call <vilib>:"Std Deviation and Variance.vi"("X"=w2992) -> ("standard deviation"=w2994:dbl)  [unwired: 1 in, 2 out]
    n2297 = Build Array(w3139, w3138, w2982) -> (→"APD Chart":waveform(dbl)[])
    n2298 = Divide(x=w2995, y=w2993) -> (x/y=w2989:dbl)
    "APD 3 Rate (Hz)" <- w2989
    n2299 = Divide(x=w2994, y=w2991) -> (x/y=w2990:dbl)
    "Rate sigma (Hz) 3" <- w2990
    n2300 = Divide(x=w2990, y=w2989) -> (x/y=→"Sigma/Mean 3":dbl)
    n2301 = local read "Data Period (s)"() -> (w3046:dbl)
    n2302 = local read "BD 1 Frequency 2 (MHz)"() -> (w3079:dbl)
    n2303 = local read "BD 1 Frequency 1 (MHz)"() -> (w3080:dbl)
    n2304 = Decimate 1D Array(w3087) -> (w3111:i16[], w3110:i16[], w3108:i16[], w3107:i16[])  [unwired: 9 out]
    n2305 = Multiply(x=w3046, y="Trap Pos. Disp. Downsample") -> (x*y=w3044:dbl)
    n2306 = Divide(x=w3111, y=w3110) -> (x/y=w3112:dbl[])
    n2307 = Divide(x=w3108, y=w3107) -> (x/y=w3109:dbl[])
    n2308 = local read "AOM X Cal (nm/MHz)"() -> (w3077:dbl)
    n2309 = Split 1D Array(array=w3112, index="N El. to Ave.") -> (second subarray=w3115:dbl[])  [unwired: 1 out]
    n2310 = Split 1D Array(array=w3109, index="N El. to Ave.") -> (second subarray=w3114:dbl[])  [unwired: 1 out]
    n2311 = Multiply(x=w3046, y="Trap Disp. Downsample") -> (x*y=w3125:dbl)
    "Display Period (s)" <- w3125
    n2312 = for "Trap AI" {
      tunnel: [w3908] -> w3290 mode=indexing
      tunnel: w3123 -> [w3899]
      tunnel: "Trap Disp. Downsample" -> [w3906]
      tunnel: w3189 -> [w3904] mode=indexing
      tunnel: w3046 -> [w3903]
      tunnel: w3188 -> [w3902] mode=indexing
      tunnel: [w3901] -> w3158 mode=indexing
      tunnel: w3125 -> [w3900]
      workers-P: _ -> [_]
      n2313 = Bundle By Name("Y"=w3904, "dt"=w3903) -> (w3905:waveform(dbl))  [unwired: 1 out]
      n2314 = Set Waveform Attribute(5:w3902, 6:"NI_ChannelName" ("name"), 7:w3905) -> (3:w3901:waveform(dbl))  [unwired: 1 in, 2 out]
      n2315 = call "downsample 1D array - double.vi"("Ave N"=w3906, "Array In"=w3904) -> ("Array Out"=w3907:dbl[])  [unwired: 1 out]
      n2316 = Bundle By Name(cluster=w3901, "t0"=w3899, "Y"=w3907, "dt"=w3900) -> (w3908:waveform(dbl))
    }
    n2317 = Bundle("BD 1 Frequency 1 (MHz)"=w3080, "BD 1 Frequency 2 (MHz)"=w3079) -> (w3081:T42)  [unwired: 1 out]
    n2318 = call-poly <vilib>:"Mean.vi"("X"=w3114) -> ("mean"=w3102:dbl)  [unwired: 1 out]
    n2319 = call-poly <vilib>:"Mean.vi"("X"=w3115) -> ("mean"=w3103:dbl)  [unwired: 1 out]
    n2320 = Reciprocal(x=w3125) -> (1/x=→"Trap Disp. Freq. (Hz)":dbl)
    n2321 = Cluster To Array(cluster=w3081) -> (array=w3078:dbl[])
    n2322 = local read "Trap X AI1 (DMA)"() -> (w3113:T13)
    n2323 = local read "Data points/scans (MCL)"() -> (w3268:dbl)
    n2324 = To Fixed-Point(number=w3102) -> (fixed-point=w3100:fxp<+/-,16,1>)  [unwired: 1 in]
    n2325 = To Fixed-Point(number=w3103) -> (fixed-point=w3101:fxp<+/-,16,1>)  [unwired: 1 in]
    n2326 = Bundle("Trap 1 Pos.", "Trap 2 Pos.") -> (w3122:cluster{string, string})  [unwired: 1 out]
    n2327 = Bundle By Name(cluster=w3113, "Set 1"=w3101, "Set 2"=w3100) -> (→"Trap X AI1 (DMA)":T13)
    n2328 = Cluster To Array(cluster=w3122) -> (array=w3119:string[])
    n2329 = Unbundle(w2977) -> (w2978:u32[])  [unwired: 2 out]
    n2330 = Select(t=-1.0, s="Negate Y Axis", f=1.0) -> (s? t:f=w3063:dbl)
    n2331 = for "Trap Position" {
      tunnel: w3127 -> [w3494] mode=indexing
      tunnel: "Trap Pos. Disp. Downsample" -> [w3493]
      tunnel: w3044 -> [w3491]
      tunnel: w3123 -> [w3490]
      tunnel: w3119 -> [w3488] mode=indexing
      tunnel: [w3487] -> w3033 mode=indexing
      tunnel: w3078 -> [w3485] mode=indexing
      tunnel: w3077 -> [w3483]
      tunnel: w3063 -> [w3482]
      n2332 = call "downsample 1D array - double.vi"("Ave N"=w3493, "Array In"=w3494) -> ("Array Out"=w3492:dbl[])  [unwired: 1 out]
      n2333 = Subtract(x=w3492, y=w3485) -> (x-y=w3486:dbl[])
      n2334 = Multiply(x=w3483, y=w3486) -> (x*y=w3484:dbl[])
      n2335 = Multiply(x=w3482, y=w3484) -> (x*y=w3481:dbl[])
      n2336 = Bundle By Name("Y"=w3481, "dt"=w3491, "t0"=w3490) -> (w3489:waveform(dbl))  [unwired: 1 out]
      n2337 = Set Waveform Attribute(5:w3488, 6:"NI_ChannelName" ("name"), 7:w3489) -> (3:w3487:waveform(dbl))  [unwired: 1 in, 2 out]
    }
    n2338 = To Double Precision Float(number=w2978) -> (double precision float=w3186:dbl[])
    n2339 = local read "Display Period (s)"() -> (w3175:dbl)
    n2340 = Increment(x=w3268) -> (x+1=w3269:dbl)
    n2341 = Index Array(array=w3033, index=0) -> (element=w3037:waveform(dbl))
    n2342 = Index Array(array=w3033, index=1) -> (element=w3032:waveform(dbl))
    n2343 = feedback #7(w3269) -> (w3272:dbl)
    n2344 = Select(t=0, s=w3259, f=w3272) -> (s? t:f=w3265:dbl)
    n2345 = Array Size(array=w3186) -> (size(s)=w3271:i32)
    n2346 = Build Array (concatenate)(w3154, w3290) -> (w3156:waveform(dbl)[])
    "All Signals" <- w3156
    n2347 = Add(x=w3271, y=w3265) -> (x+y=w3266:dbl)
    n2348 = Unbundle By Name(w3037) -> ("Y"=w3038:dbl[])
    n2349 = Divide(x="Bead Sep. Int. Time (s)", y=w3175) -> (x/y=w3073:dbl)
    n2350 = Add(x=w3038, y="FB Trap Pos Offset") -> (x+y=w3036:dbl[])
    "T1 x pos data" <- w3036
    n2351 = Greater?(x=w3266, y=w3268) -> (0:w3267:bool)
    n2352 = feedback #8(w3036) -> (w3075:dbl[])
    n2353 = Build Array (concatenate)(w3036, w3075) -> (w3074:dbl[])
    n2354 = Bundle By Name(cluster=w3037, "Y"=w3036) -> (w3035:waveform(dbl))
    n2355 = Select(t=w3265, s=w3267, f=w3266) -> (s? t:f=w3264:dbl)
    n2356 = feedback-in #7(w3264) -> ()
    n2357 = local read "MCL Scanning"() -> (w3262:bool)
    n2358 = Bundle(w3035, w3032) -> (w3031:cluster{waveform(dbl), waveform(dbl)})  [unwired: 1 out]
    n2359 = Split 1D Array(array=w3074, index=w3073) -> (first subarray=w3067:dbl[])  [unwired: 1 out]
    n2360 = feedback-in #8(w3067) -> ()
    n2361 = Not(x=w3267) -> (.not. x?=w3261:bool)
    n2362 = Cluster To Array(cluster=w3031) -> (array=w3007:waveform(dbl)[])
    "Trap Positions" <- w3007
    n2363 = call-poly <vilib>:"Mean.vi"("X"=w3067) -> ("mean"=w3066:dbl)  [unwired: 1 out]
    "Mean T1 Position (nm)" <- w3066
    n2364 = Subtract(x=w3067, y=w3066) -> (x-y=w3072:dbl[])
    n2365 = Square(x=w3072) -> (x^2=w3071:dbl[])
    n2366 = And(x=w3261, y=w3262) -> (x .and. y?=w3263:bool)
    n2367 = call-poly <vilib>:"Mean.vi"("X"=w3071) -> ("mean"=w3070:dbl)  [unwired: 1 out]
    n2368 = Square Root(x=w3070) -> (sqrt(x)=w3069:dbl)
    n2369 = Or(x=w3263, y=w3259) -> (x .or. y?=w3260:bool)
    n2370 = Equal?(x="Tab Control 6", y=T32."High Res Display") -> (x = y?=w3192:bool)
    n2371 = Multiply(x=10.0, y=w3069) -> (x*y=→"Trap 1 Position RMS (A)":dbl)
    n2372 = case "For displaying the high resolution display (no downsampling)" shown="True" w3192 {
      tunnel: w3158 -> [_ w3514]
      frame False {
      }
      frame True {
        n2373 = Index Array(array=w3514, index="High Res. Display") -> (element=w3515:waveform(dbl))
        n2374 = call <vilib>:"Std Deviation and Variance.vi"("X"=w3515) -> ("mean"=w3522:dbl, "standard deviation"=w3527:dbl)  [unwired: 1 in, 1 out]
        "Mean Intensity" <- w3522
        "Sigma" <- w3527
        n2375 = Subtract(x=w3515, y=w3522) -> (x-y=w3521:waveform(dbl))
        n2376 = Select(t=w3521, s="Subtract mean", f=w3515) -> (s? t:f=→"1 Channel":waveform(dbl))
        n2377 = Divide(x=w3527, y=w3522) -> (x/y=→"Sigma/Mean":dbl)
        n2378 = feedback #9(1) -> (w3516:i32)
        n2379 = Greater Or Equal?(x=w3516, y="Slow mean N ave.") -> (x >= y?=w3529:bool)
        n2380 = Increment(x=w3516) -> (x+1=w3531:i32)
        n2381 = Select(t=1, s=w3529, f=w3531) -> (s? t:f=w3518:i32)
        n2382 = feedback-in #9(w3518) -> ()
        n2383 = feedback #10() -> (w3519:waveform(dbl))  [unwired: 1 out]
        n2384 = case shown="Default" w3516 {
          tunnel: [w3534 w3537] -> w3520
          tunnel: w3519 -> [w3536 _]
          tunnel: w3515 -> [w3535 w3537]
          frame Default {
            n2385 = call-poly <vilib>:"Append Waveforms.vi"("waveform B"=w3535, "waveform A"=w3536) -> ("waveform out"=w3534:waveform(dbl))  [unwired: 1 in, 8 out]
          }
          frame 1 {
          }
        }
        n2386 = feedback-in #10(w3520) -> ()
        n2387 = case shown="True" w3529 {
          tunnel: w3520 -> [_ w3533]
          frame False {
          }
          frame True {
            n2388 = call-poly <vilib>:"Mean.vi"("X"=w3533) -> ("mean"=→"Slow mean":dbl)  [unwired: 1 out]
          }
        }
      }
    }
    n2389 = case "For plotting results of scanning MCL (fluorescence and detection laser images)" shown="True" w3260 {
      tunnel: w3259 -> [_ w3646]
      tunnel: w3268 -> [_ _]
      tunnel: w3158 -> [_ w3776]
      tunnel: w3136 -> [_ w3684]
      tunnel: w2977 -> [_ w3653]
      frame False {
      }
      frame True {
        w3663 = u32 0 items=["Horizontal", "Vertical", "Central", "1st Diagonal", "2nd Diagonal"] ("Type of Symmetry")
        w3691 = u32 0 items=["Horizontal", "Vertical", "Central", "1st Diagonal", "2nd Diagonal"] ("Type of Symmetry")
        w3715 = u32 0 items=["Horizontal", "Vertical", "Central", "1st Diagonal", "2nd Diagonal"] ("Type of Symmetry")
        w3718 = u32 0 items=["Horizontal", "Vertical", "Central", "1st Diagonal", "2nd Diagonal"] ("Type of Symmetry")
        w3747 = u32 0 items=["Horizontal", "Vertical", "Central", "1st Diagonal", "2nd Diagonal"] ("Type of Symmetry")
        n2390 = Unbundle(w3653) -> (w3652:u32[], w3650:u32[], w3648:u32[])
        n2391 = To Double Precision Float(number=w3652) -> (double precision float=w3651:dbl[])
        n2392 = To Double Precision Float(number=w3650) -> (double precision float=w3649:dbl[])
        n2393 = To Double Precision Float(number=w3648) -> (double precision float=w3647:dbl[])
        n2394 = Index Array(array=w3776, index=10) -> (element=w3782:waveform(dbl))
        n2395 = Index Array(array=w3776, index=11) -> (element=w3779:waveform(dbl))
        n2396 = local read "Cycles/step (MCL)"() -> (w3732:u64)
        n2397 = Index Array(array=w3776, index="Channel") -> (element=w3778:waveform(dbl))
        n2398 = Unbundle(w3684) -> ("New Image"=w3683:T2, "New Image"=w3682:T2, "New Image"=w3654:T2, "New Image"=w3655:T2, "New Image"=w3656:T2)
        n2399 = local read "Scan steps (MCL)"() -> (w3642:u64)
        n2400 = Unbundle By Name(w3782) -> ("Y"=w3734:dbl[])
        n2401 = Unbundle By Name(w3779) -> ("Y"=w3736:dbl[])
        n2402 = local read "Scan lines (y)"() -> (w3643:u64)
        n2403 = local read "N APD Samp/step"() -> (w3645:dbl)
        n2404 = Unbundle By Name(w3778) -> ("Y"=w3741:dbl[])
        n2405 = call "downsample 1D array - double.vi"("Ave N"=w3732, "Array In"=w3734) -> ("Array Out"=w3733:dbl[])  [unwired: 1 out]
        n2406 = call "downsample 1D array - double.vi"("Ave N"=w3732, "Array In"=w3736) -> ("Array Out"=w3735:dbl[])  [unwired: 1 out]
        n2407 = call "downsample 1D array - double.vi"("Ave N"=w3732, "Array In"=w3741) -> ("Array Out"=w3740:dbl[])  [unwired: 1 out]
        n2408 = Multiply(x=w3642, y=u64 2) -> (x*y=w3644:u64)
        n2409 = feedback #11(w3649) -> (w3709:dbl[])
        n2410 = Build Array (concatenate)(w3709, w3649) -> (w3708:dbl[])
        n2411 = feedback #12(w3647) -> (w3681:dbl[])
        n2412 = Build Array (concatenate)(w3681, w3647) -> (w3680:dbl[])
        n2413 = Select(t=w3649, s=w3646, f=w3708) -> (s? t:f=w3693:dbl[])
        n2414 = feedback-in #11(w3693) -> ()
        n2415 = Select(t=w3647, s=w3646, f=w3680) -> (s? t:f=w3665:dbl[])
        n2416 = feedback-in #12(w3665) -> ()
        n2417 = feedback #13(w3651) -> (w3802:dbl[])
        n2418 = Build Array (concatenate)(w3802, w3651) -> (w3784:dbl[])
        n2419 = Select(t=w3651, s=w3646, f=w3784) -> (s? t:f=w3788:dbl[])
        n2420 = feedback-in #13(w3788) -> ()
        n2421 = feedback #14(w3733) -> (w3790:dbl[])
        n2422 = Build Array (concatenate)(w3790, w3733) -> (w3781:dbl[])
        n2423 = feedback #15(w3740) -> (w3800:dbl[])
        n2424 = Build Array (concatenate)(w3800, w3740) -> (w3799:dbl[])
        n2425 = feedback #16(w3735) -> (w3792:dbl[])
        n2426 = Build Array (concatenate)(w3792, w3735) -> (w3793:dbl[])
        n2427 = Select(t=w3733, s=w3646, f=w3781) -> (s? t:f=w3737:dbl[])
        n2428 = feedback-in #14(w3737) -> ()
        n2429 = Select(t=w3740, s=w3646, f=w3799) -> (s? t:f=w3739:dbl[])
        n2430 = feedback-in #15(w3739) -> ()
        n2431 = Select(t=w3735, s=w3646, f=w3793) -> (s? t:f=w3738:dbl[])
        n2432 = feedback-in #16(w3738) -> ()
        n2433 = call "integrate 1D array interval - double.vi"("Ave N"=w3645, "Array In"=w3693) -> ("Array Out"=w3704:dbl[])  [unwired: 1 out]
        n2434 = call "integrate 1D array interval - double.vi"("Ave N"=w3645, "Array In"=w3665) -> ("Array Out"=w3676:dbl[])  [unwired: 1 out]
        n2435 = call "integrate 1D array interval - double.vi"("Ave N"=w3645, "Array In"=w3788) -> ("Array Out"=w3787:dbl[])  [unwired: 1 out]
        n2436 = Array Size(array=w3704) -> (size(s)=w3705:i32)
        n2437 = Array Size(array=w3676) -> (size(s)=w3677:i32)
        n2438 = Array Size(array=w3787) -> (size(s)=w3789:i32)
        n2439 = Multiply(x=w3643, y=w3644) -> (x*y=w3707:u64)
        n2440 = Multiply(x=w3643, y=w3644) -> (x*y=w3679:u64)
        n2441 = Multiply(x=w3643, y=w3644) -> (x*y=w3797:u64)
        n2442 = Subtract(x=w3707, y=w3705) -> (x-y=w3698:u64)
        n2443 = call-poly <vilib>:"Mean.vi"("X"=w3704) -> ("mean"=w3695:dbl)  [unwired: 1 out]
        n2444 = Subtract(x=w3679, y=w3677) -> (x-y=w3670:u64)
        n2445 = call-poly <vilib>:"Mean.vi"("X"=w3676) -> ("mean"=w3667:dbl)  [unwired: 1 out]
        n2446 = Subtract(x=w3797, y=w3789) -> (x-y=w3731:u64)
        n2447 = call-poly <vilib>:"Mean.vi"("X"=w3787) -> ("mean"=w3728:dbl)  [unwired: 1 out]
        n2448 = call-poly <vilib>:"Mean.vi"("X"=w3737) -> ("mean"=w3721:dbl)  [unwired: 1 out]
        n2449 = call-poly <vilib>:"Mean.vi"("X"=w3739) -> ("mean"=w3726:dbl)  [unwired: 1 out]
        n2450 = call-poly <vilib>:"Mean.vi"("X"=w3738) -> ("mean"=w3724:dbl)  [unwired: 1 out]
        n2451 = Initialize Array(1.0 ("element"), w3698) -> (w3694:dbl[])
        n2452 = Initialize Array(1.0 ("element"), w3670) -> (w3666:dbl[])
        n2453 = Initialize Array(1.0 ("element"), w3731) -> (w3722:dbl[])
        n2454 = Multiply(x=w3694, y=w3695) -> (x*y=w3696:dbl[])
        n2455 = Multiply(x=w3666, y=w3667) -> (x*y=w3668:dbl[])
        n2456 = Multiply(x=w3722, y=w3728) -> (x*y=w3729:dbl[])
        n2457 = Multiply(x=w3722, y=w3724) -> (x*y=w3725:dbl[])
        n2458 = Multiply(x=w3722, y=w3726) -> (x*y=w3727:dbl[])
        n2459 = Multiply(x=w3722, y=w3721) -> (x*y=w3723:dbl[])
        n2460 = Build Array (concatenate)(w3704, w3696) -> (w3706:dbl[])
        n2461 = Build Array (concatenate)(w3676, w3668) -> (w3678:dbl[])
        n2462 = Build Array (concatenate)(w3787, w3729) -> (w3796:dbl[])
        n2463 = Build Array (concatenate)(w3737, w3723) -> (w3791:dbl[])
        n2464 = Build Array (concatenate)(w3739, w3727) -> (w3795:dbl[])
        n2465 = Build Array (concatenate)(w3738, w3725) -> (w3794:dbl[])
        n2466 = Reshape Array(w3706, w3643, w3644) -> (w3702:dbl[][])
        n2467 = Reshape Array(w3678, w3643, w3644) -> (w3674:dbl[][])
        n2468 = Reshape Array(w3796, w3643, w3644) -> (w3774:dbl[][])
        n2469 = Reshape Array(w3791, w3643, w3644) -> (w3757:dbl[][])
        n2470 = Reshape Array(w3795, w3643, w3644) -> (w3749:dbl[][])
        n2471 = Reshape Array(w3794, w3643, w3644) -> (w3764:dbl[][])
        n2472 = Array Subset(array=w3702, index (col)=0 ("index"), length (col)=w3642) -> (w3701:dbl[][])  [unwired: 2 in]
        n2473 = Array Subset(array=w3702, index (col)=w3642) -> (w3699:dbl[][])  [unwired: 3 in]
        n2474 = Array Subset(array=w3674, index (col)=0 ("index"), length (col)=w3642) -> (w3673:dbl[][])  [unwired: 2 in]
        n2475 = Array Subset(array=w3674, index (col)=w3642) -> (w3671:dbl[][])  [unwired: 3 in]
        n2476 = Array Subset(array=w3764, index (col)=0 ("index"), length (col)=w3642) -> (w3769:dbl[][])  [unwired: 2 in]
        n2477 = Array Subset(array=w3764, index (col)=w3642) -> (w3767:dbl[][])  [unwired: 3 in]
        n2478 = Array Subset(array=w3774, index (col)=0 ("index"), length (col)=w3642) -> (w3773:dbl[][])  [unwired: 2 in]
        n2479 = Array Subset(array=w3774, index (col)=w3642) -> (w3771:dbl[][])  [unwired: 3 in]
        n2480 = Array Subset(array=w3749, index (col)=0 ("index"), length (col)=w3642) -> (w3755:dbl[][])  [unwired: 2 in]
        n2481 = Array Subset(array=w3749, index (col)=w3642) -> (w3753:dbl[][])  [unwired: 3 in]
        n2482 = Array Subset(array=w3757, index (col)=0 ("index"), length (col)=w3642) -> (w3762:dbl[][])  [unwired: 2 in]
        n2483 = Array Subset(array=w3757, index (col)=w3642) -> (w3760:dbl[][])  [unwired: 3 in]
        n2484 = for {
          tunnel: w3701 -> [w3806] mode=indexing
          tunnel: [w3805] -> w3700 mode=indexing
          workers-P: _ -> [_]
          n2485 = Reverse 1D Array(array=w3806) -> (reversed array=w3805:dbl[])
        }
        n2486 = for {
          tunnel: w3673 -> [w3804] mode=indexing
          tunnel: [w3803] -> w3672 mode=indexing
          workers-P: _ -> [_]
          n2487 = Reverse 1D Array(array=w3804) -> (reversed array=w3803:dbl[])
        }
        n2488 = for {
          tunnel: w3769 -> [w3812] mode=indexing
          tunnel: [w3811] -> w3768 mode=indexing
          workers-P: _ -> [_]
          n2489 = Reverse 1D Array(array=w3812) -> (reversed array=w3811:dbl[])
        }
        n2490 = for {
          tunnel: w3773 -> [w3814] mode=indexing
          tunnel: [w3813] -> w3772 mode=indexing
          workers-P: _ -> [_]
          n2491 = Reverse 1D Array(array=w3814) -> (reversed array=w3813:dbl[])
        }
        n2492 = for {
          tunnel: w3755 -> [w3808] mode=indexing
          tunnel: [w3807] -> w3754 mode=indexing